vi "UHR-Fleezers Control (host) - 12.7.vi"() -> ()   [LabVIEW 2012] (continued)
                                }
                                frame "4" {
                                n759 = property on="Fl. Triggered..." class="Bool (strict)"("Val(Sgnl)"=TRUE ("Value (Signaling)")) -> ()  [unwired: 2 in, 2 out]
                                }
                                }
                                }
                                }
                                }
                                frame "5", "6" {
                                n760 = stacked-sequence {
                                tunnel: w1212 -> [_ _ _ _ _ _ w1224]
                                frame #0 {
                                n761 = Replace Array Subset(array=u32[] [0] ("Index Values"), new element="Raster Set Upon Tether", index=0) -> (w1213:u32[])
                                n762 = property on="Saved AOD Raster Scan Parameter Sets" class="Arr (strict)"("Index Values"=w1213) -> ()  [unwired: 2 in, 2 out]
                                }
                                frame #1 {
                                n763 = Wait (ms)(milliseconds to wait=u32 500) -> ()  [unwired: 1 out]
                                }
                                frame #2 {
                                n764 = property on="Load parameters" class="Bool (strict)"("Val(Sgnl)"=TRUE ("Value (Signaling)")) -> ()  [unwired: 2 in, 2 out]
                                n765 = case shown="True" "Green ON During Raster" {
                                frame False {
                                }
                                frame True {
                                n766 = property on="Green Laser ON" class="Bool (strict)"("Val(Sgnl)"=TRUE ("Value (Signaling)")) -> ()  [unwired: 2 in, 2 out]
                                }
                                }
                                }
                                frame #3 {
                                n767 = Wait (ms)(milliseconds to wait=u32 500) -> ()  [unwired: 1 out]
                                }
                                frame #4 {
                                n768 = property on="Trap Raster Scan" class="Bool (strict)"("Val(Sgnl)"=TRUE ("Value (Signaling)")) -> ()  [unwired: 2 in, 2 out]
                                }
                                frame #5 {
                                n769 = Wait (ms)(milliseconds to wait=u32 2000) -> ()  [unwired: 1 out]
                                }
                                frame #6 {
                                n770 = flat-sequence {
                                tunnel: w1224 -> [w1231]
                                frame #0 {
                                n771 = while {
                                stop <- w1227 stop-if-true
                                n772 = local read "Raster Scanning..."() -> (w1226:bool)
                                n773 = local read "Saving..."() -> (w1229:bool)
                                n774 = Wait (ms)(milliseconds to wait=u32 100) -> ()  [unwired: 1 out]
                                n775 = Not(x=w1229) -> (.not. x?=w1228:bool)
                                n776 = Not(x=w1226) -> (.not. x?=w1225:bool)
                                n777 = And(x=w1228, y=w1225) -> (x .and. y?=w1227:bool)
                                }
                                }
                                frame #1 {
                                n778 = local read "Tether"() -> (w1232:bool)
                                n779 = case shown="True" w1232 {
                                tunnel: w1231 -> [_ w1234]
                                frame False {
                                n780 = property on="Fish for Tether" class="Bool (strict)"("Val(Sgnl)"="Fish again after \nraster break?") -> ()  [unwired: 2 in, 2 out]
                                }
                                frame True {
                                n781 = stacked-sequence {
                                tunnel: w1234 -> [_ w1238 _ _]
                                frame #0 {
                                n782 = property on="Trap Delta (MHz)" class="DigNum (strict)"("Val(Sgnl)"="Move to Delta 2 (MHz)") -> ()  [unwired: 2 in, 2 out]
                                n783 = case shown="True" "Flow ON after\ntether testing?" {
                                frame False {
                                }
                                frame True {
                                n784 = property on="Sample Channel\nFlow" class="Bool (strict)"("Val(Sgnl)"=TRUE ("Value (Signaling)")) -> ()  [unwired: 2 in, 2 out]
                                }
                                }
                                }
                                frame #1 {
                                n785 = flat-sequence {
                                tunnel: w1238 -> [w1240]
                                frame #0 {
                                n786 = Wait (ms)(milliseconds to wait=u32 500) -> ()  [unwired: 1 out]
                                }
                                frame #1 {
                                n787 = case shown="\"6\"" w1240 {
                                frame Default {
                                }
                                frame "6" {
                                n788 = property on="Green Laser ON" class="Bool (strict)"("Val(Sgnl)"=TRUE ("Green Laser ON/Interlacing")) -> ()  [unwired: 2 in, 2 out]
                                }
                                }
                                }
                                frame #2 {
                                n789 = Wait (ms)(milliseconds to wait=u32 500) -> ()  [unwired: 1 out]
                                }
                                frame #3 {
                                n790 = local write "Start Saving"("Save at end (5, 6)") -> ()
                                }
                                }
                                }
                                frame #2 {
                                n791 = local read "Bead Sep. Int. Time (s)"() -> (w1246:dbl)
                                n792 = Multiply(x=w1246, y=1000.0) -> (x*y=w1245:dbl)
                                n793 = Wait (ms)(milliseconds to wait=w1245) -> ()  [unwired: 1 out]
                                }
                                frame #3 {
                                n794 = property on="Remove Offset" class="Bool (strict)"("Val(Sgnl)"=TRUE ("Value (Signaling)")) -> ()  [unwired: 2 in, 2 out]
                                }
                                }
                                }
                                }
                                }
                                }
                                }
                                }
                                }
                                frame "2", Default {
                                }
                              }
                            }
                          }
                        }
                      }
                      "Tether" <- "Tether Alarm?"
                    }
                  }
                }
                frame #2 {
                  n795 = local read "Oscillate Set 1"() -> (w1253:bool)
                  n796 = local read "Stop All"() -> (w1251:bool)
                  n797 = Or(x=w1253, y=w1248) -> (x .or. y?=w1250:bool)
                  n798 = Not(x=w1250) -> (.not. x?=w1252:bool)
                  n799 = Compound Arithmetic op=OR(w1251, w1252) -> (w1249:bool)
                }
              }
              n800 = node-c288() -> ()  [unwired: 2 out]
            }
            n801 = node-c288(w1085) -> ()  [unwired: 1 out]
          }
        }
      }
      event "Fl. Triggered...": Value Change {
        n802 = event-data() -> ()  [unwired: 7 out]
        n803 = case shown="True" "Fl. Triggered..." {
          frame False {
          }
          frame True {
            n804 = node-c288() -> (w1264:T23)  [unwired: 4 out]
            n805 = timed-loop {
              timing: w1264 -> [_]
              timing-out: [_] -> w1263
              tunnel: "Action" -> [w1272]
              shift-right: [w1269] -> _
              shift-left: u8 255 -> [w1271]
              shift-right: [w1266] -> _
              shift-left: 255 -> [w1268]
              stop <- w1265 stop-if-true
              # "Reset confocal spot"
              n806 = node-c288() -> ()  [unwired: 2 out]
              n807 = flat-sequence {
                tunnel: w1272 -> [w1292]
                tunnel: w1271 -> [w1291]
                tunnel: [w1290] -> w1270
                tunnel: w1268 -> [w1277]
                tunnel: [w1276] -> w1267
                tunnel: [w1671] -> w1265
                tunnel: w1270 -> [w1670]
                tunnel: [w1670] -> w1269
                tunnel: [w1669] -> w1266
                tunnel: w1267 -> [w1669]
                frame #0 {
                  n808 = local read "Delta Fl. 2"() -> (w1289:dbl)
                  n809 = local read "Delta Fl. 1"() -> (w1284:dbl)
                  n810 = Multiply(x="Fl. Delta Thresh. (kHz)", y=1000.0) -> (x*y=w1279:dbl)
                  n811 = Select(t=w1284, s="APD to Watch", f=w1289) -> (s? t:f=w1280:dbl)
                  n812 = Greater?(x=w1280, y=w1279) -> (0:w1285:bool)
                  n813 = Or(x="Force Yank", y=w1285) -> (x .or. y?=w1283:bool)
                  n814 = And(x=w1283, y="Yank when?") -> (x .and. y?=w1281:bool)
                  n815 = case shown="False" w1281 {
                    tunnel: w1292 -> [w1295 w1496]
                    tunnel: w1291 -> [w1297 w1492]
                    tunnel: [w1297 w1490] -> w1290
                    tunnel: w1280 -> [w1303 _]
                    tunnel: w1279 -> [w1302 _]
                    tunnel: "Force Yank" -> [w1300 _]
                    tunnel: w1277 -> [w1299 w1489]
                    tunnel: [w1298 w1489] -> w1276
                    frame False {
                      n816 = Negate(x=w1302) -> (-x=w1294:dbl)
                      n817 = local write "Fl. High"(TRUE ("Fl. High")) -> ()
                      n818 = Less?(x=w1303, y=w1294) -> (x < y?=w1301:bool)
                      n819 = Or(x=w1300, y=w1301) -> (x .or. y?=w1296:bool)
                      n820 = case shown="True" w1296 {
                        tunnel: w1299 -> [w1304 w1314]
                        tunnel: [w1304 w1313] -> w1298
                        tunnel: w1295 -> [_ w1312]
                        frame False {
                        }
                        frame True {
                          n821 = flat-sequence {
                            tunnel: w1314 -> [w1320]
                            tunnel: w1312 -> [w1317]
                            tunnel: [w1319] -> w1311
                            tunnel: [w1318] -> w1310
                            tunnel: [w1317] -> w1309
                            tunnel: w1308 -> [w1316]
                            tunnel: [w1316] -> w1307
                            tunnel: w1306 -> [w1315]
                            tunnel: [w1315] -> w1305
                            tunnel: [w1391] -> w1313
                            tunnel: w1311 -> [w1391]
                            tunnel: w1310 -> [w1390]
                            tunnel: w1309 -> [w1389]
                            tunnel: w1307 -> [w1388]
                            tunnel: w1305 -> [w1387]
                            frame #0 {
                              n822 = call <vilib>:"Beep.vi"() -> ()  [unwired: 12 in]
                              n823 = local write "Waiting"(FALSE ("Waiting")) -> ()
                              n824 = Increment(x=w1320) -> (x+1=w1319:i32)
                              n825 = case shown="\"Image\"" w1317 {
                                tunnel: w1319 -> [_ w1325 _]
                                frame "Alarm", Default {
                                }
                                frame "Yank" {
                                n826 = flat-sequence {
                                tunnel: w1325 -> [w1328]
                                tunnel: [w1327] -> w1324
                                tunnel: [w1326] -> w1323
                                tunnel: w1324 -> [w1338]
                                tunnel: w1323 -> [w1339]
                                frame #0 {
                                n827 = local read "Yank Delay (s)"() -> (w1331:dbl)
                                n828 = local read "N Array El"() -> (w1326:u8)
                                n829 = Quotient & Remainder(x=w1328, y=w1326) -> (x-y*floor(x/y)=w1327:i32)  [unwired: 1 out]
                                n830 = Multiply(x=w1331, y=1000.0) -> (x*y=w1329:dbl)
                                n831 = Wait (ms)(milliseconds to wait=w1329) -> ()  [unwired: 1 out]
                                }
                                frame #1 {
                                n832 = local read "Yank to which?"() -> (w1333:bool)
                                n833 = local read "Random Choice"() -> (w1343:bool)
                                n834 = local read "Yank to Trap Delta (MHz)"() -> (w1336:dbl[])
                                n835 = local read "Yank to SP"() -> (w1337:dbl[])
                                n836 = Random Number (0-1)() -> (number: 0 to 1=w1342:dbl)
                                n837 = Multiply(x=w1339, y=w1342) -> (x*y=w1341:dbl)
                                n838 = Round Toward -Infinity(1:w1341) -> (0:w1340:dbl)
                                n839 = Select(t=w1340, s=w1343, f=w1338) -> (s? t:f=w1334:dbl)
                                n840 = Select(t=w1336, s=w1333, f=w1337) -> (s? t:f=w1335:dbl[])
                                n841 = Index Array(array=w1335, index=w1334) -> (element=w1332:dbl)
                                n842 = case shown="True" w1333 {
                                tunnel: w1332 -> [w1344 w1371]
                                frame False {
                                n843 = flat-sequence {
                                tunnel: w1344 -> [w1345]
                                frame #0 {
                                n844 = property on="Trap Pos FB SP" class="DigNum (strict)"("Val(Sgnl)"=w1345) -> ()  [unwired: 2 in, 2 out]
                                }
                                frame #1 {
                                n845 = Wait (ms)(milliseconds to wait=u32 700) -> ()  [unwired: 1 out]
                                }
                                frame #2 {
                                n846 = local read "Action (%)"() -> (w1350:dbl)
                                n847 = Absolute Value(x=w1350) -> (abs(x)=w1349:dbl)
                                n848 = Greater?(x=w1349, y=70.0) -> (0:w1347:bool)
                                n849 = property on="Remove Action Offset" class="Bool (strict)"("Val(Sgnl)"=w1347) -> ()  [unwired: 2 in, 2 out]
                                }
                                frame #3 {
                                n850 = for {
                                N: 4 -> [_]
                                n851 = flat-sequence {
                                frame #0 {
                                n852 = Wait (ms)(milliseconds to wait=u32 500) -> ()  [unwired: 1 out]
                                }
                                frame #1 {
                                n853 = local read "Action (%)"() -> (w1356:dbl)
                                n854 = Absolute Value(x=w1356) -> (abs(x)=w1355:dbl)
                                n855 = Greater?(x=w1355, y=70.0) -> (0:w1353:bool)
                                n856 = property on="Remove Action Offset" class="Bool (strict)"("Val(Sgnl)"=w1353) -> ()  [unwired: 2 in, 2 out]
                                }
                                }
                                }
                                }
                                frame #4 {
                                n857 = Wait (ms)(milliseconds to wait=u32 500) -> ()  [unwired: 1 out]
                                }
                                frame #5 {
                                n858 = local read "Mean"() -> (w1364:dbl)
                                n859 = Greater?(x=w1364, y=11.0) -> (0:w1358:bool)
                                n860 = Not(x=w1358) -> (.not. x?=w1359:bool)
                                n861 = And(x=w1359, y="Shift confocal") -> (x .and. y?=w1361:bool)
                                n862 = And(x=w1358, y="Shift confocal") -> (x .and. y?=w1362:bool)
                                n863 = case shown="True" w1362 {
                                frame False {
                                }
                                frame True {
                                n864 = local read "Confocal Y 2 (V)"() -> (w1368:dbl)
                                n865 = local read "Confocal X 2 (V)"() -> (w1367:dbl)
                                n866 = property on="AO1" class="Slide (strict)"("Val(Sgnl)"=w1368) -> ()  [unwired: 2 in, 2 out]
                                n867 = property on="AO2" class="Slide (strict)"("Val(Sgnl)"=w1367) -> ()  [unwired: 2 in, 2 out]
                                }
                                }
                                n868 = case shown="True" w1361 {
                                frame False {
                                }
                                frame True {
                                n869 = local read "Confocal Y 1 (V)"() -> (w1366:dbl)
                                n870 = local read "Confocal X 1 (V)"() -> (w1365:dbl)
                                n871 = property on="AO1" class="Slide (strict)"("Val(Sgnl)"=w1366) -> ()  [unwired: 2 in, 2 out]
                                n872 = property on="AO2" class="Slide (strict)"("Val(Sgnl)"=w1365) -> ()  [unwired: 2 in, 2 out]
                                }
                                }
                                }
                                frame #6 {
                                n873 = Wait (ms)(milliseconds to wait=u32 1500) -> ()  [unwired: 1 out]
                                }
                                frame #7 {
                                n874 = property on="Rem fb disp offset" class="Bool (strict)"("Val(Sgnl)"=TRUE ("Value (Signaling)")) -> ()  [unwired: 2 in, 2 out]
                                }
                                }
                                }
                                frame True {
                                n875 = flat-sequence {
                                tunnel: w1371 -> [w1372]
                                frame #0 {
                                n876 = property on="Trap Delta (MHz)" class="DigNum (strict)"("Val(Sgnl)"=w1372) -> ()  [unwired: 2 in, 2 out]
                                }
                                frame #1 {
                                n877 = Wait (ms)(milliseconds to wait=u32 500) -> ()  [unwired: 1 out]
                                }
                                frame #2 {
                                n878 = local read "Shift confocal"() -> (w1378:bool)
                                n879 = local read "Mean"() -> (w1380:dbl)
                                n880 = Greater?(x=w1380, y=11.0) -> (0:w1377:bool)
                                n881 = Not(x=w1377) -> (.not. x?=w1376:bool)
                                n882 = And(x=w1376, y=w1378) -> (x .and. y?=w1374:bool)
                                n883 = And(x=w1377, y=w1378) -> (x .and. y?=w1375:bool)
                                n884 = case shown="True" w1375 {
                                frame False {
                                }
                                frame True {
                                n885 = local read "Confocal Y 2 (V)"() -> (w1384:dbl)
                                n886 = local read "Confocal X 2 (V)"() -> (w1383:dbl)
                                n887 = property on="AO2" class="Slide (strict)"("Val(Sgnl)"=w1383) -> ()  [unwired: 2 in, 2 out]
                                n888 = property on="AO1" class="Slide (strict)"("Val(Sgnl)"=w1384) -> ()  [unwired: 2 in, 2 out]
                                }
                                }
                                n889 = case shown="True" w1374 {
                                frame False {
                                }
                                frame True {
                                n890 = local read "Confocal X 1 (V)"() -> (w1381:dbl)
                                n891 = local read "Confocal Y 1 (V)"() -> (w1382:dbl)
                                n892 = property on="AO2" class="Slide (strict)"("Val(Sgnl)"=w1381) -> ()  [unwired: 2 in, 2 out]
                                n893 = property on="AO1" class="Slide (strict)"("Val(Sgnl)"=w1382) -> ()  [unwired: 2 in, 2 out]
                                }
                                }
                                }
                                }
                                }
                                }
                                }
                                }
                                }
                                frame "Image" {
                                n894 = property on="Confocal Image" class="Bool (strict)"("Val(Sgnl)"=TRUE ("Value (Signaling)")) -> ()  [unwired: 2 in, 2 out]
                                }
                              }
                              n895 = local write "Fl. High"(FALSE ("Fl. High")) -> ()
                              n896 = local read "Time (s)"() -> (w1318:dbl)
                            }
                            frame #1 {
                              n897 = case shown="True" "Auto F Reset" {
                                tunnel: w1390 -> [_ w1395]
                                tunnel: w1389 -> [_ w1394]
                                tunnel: w1388 -> [_ w1393]
                                tunnel: w1387 -> [_ w1392]
                                frame False {
                                }
                                frame True {
                                n898 = node-c288() -> (w1397:T23)  [unwired: 4 in]
                                n899 = timed-loop {
                                timing: w1397 -> [_]
                                timing-out: [_] -> w1396
                                tunnel: w1395 -> [w1402]
                                tunnel: w1394 -> [w1401]
                                tunnel: w1393 -> [w1400]
                                tunnel: w1392 -> [w1399]
                                stop <- w1398 stop-if-true
                                n900 = node-c288() -> ()  [unwired: 1 in, 1 out]
                                n901 = local read "Fl. Delta Thresh. (kHz)"() -> (w1411:dbl)
                                n902 = local read "APD to Watch"() -> (w1412:bool)
                                n903 = local read "Delta Fl. 1"() -> (w1413:dbl)
                                n904 = local read "Delta Fl. 2"() -> (w1414:dbl)
                                n905 = local read "Fl. Triggered..."() -> (w1405:bool)
                                n906 = local read "Stop All"() -> (w1406:bool)
                                n907 = local read "Reset Force"() -> (w1404:bool)
                                n908 = Multiply(x=w1411, y=1000.0) -> (x*y=w1409:dbl)
                                n909 = Select(t=w1413, s=w1412, f=w1414) -> (s? t:f=w1408:dbl)
                                n910 = Not(x=w1405) -> (.not. x?=w1403:bool)
                                n911 = Greater?(x=w1408, y=w1409) -> (0:w1407:bool)
                                n912 = Compound Arithmetic op=OR(w1407, w1406, w1403, w1404) -> (w1398:bool)
                                n913 = case shown="True" w1398 {
                                tunnel: w1402 -> [_ w1418]
                                tunnel: w1401 -> [_ w1422]
                                tunnel: w1400 -> [_ w1421]
                                tunnel: w1399 -> [_ w1420]
                                frame False {
                                }
                                frame True {
                                n914 = case shown="\"Yank\"" w1422 {
                                tunnel: w1421 -> [_ w1432]
                                tunnel: w1420 -> [_ w1430]
                                frame "Image", Default {
                                }
                                frame "Yank" {
                                n915 = flat-sequence {
                                tunnel: [w1435] -> w1433
                                tunnel: w1432 -> [w1435]
                                tunnel: [w1434] -> w1431
                                tunnel: w1430 -> [w1434]
                                tunnel: w1433 -> [w1441]
                                tunnel: w1431 -> [w1439]
                                frame #0 {
                                n916 = local read "Yank Delay (s)"() -> (w1438:dbl)
                                n917 = Multiply(x=w1438, y=1000.0) -> (x*y=w1436:dbl)
                                n918 = Wait (ms)(milliseconds to wait=w1436) -> ()  [unwired: 1 out]
                                }
                                frame #1 {
                                n919 = local read "Yank to which?"() -> (w1440:bool)
                                n920 = case shown="False" w1440 {
                                tunnel: w1441 -> [_ w1469]
                                tunnel: w1439 -> [w1442 _]
                                frame False {
                                n921 = flat-sequence {
                                tunnel: w1442 -> [w1443]
                                frame #0 {
                                n922 = property on="Trap Pos FB SP" class="DigNum (strict)"("Val(Sgnl)"=w1443) -> ()  [unwired: 2 in, 2 out]
                                }
                                frame #1 {
                                n923 = Wait (ms)(milliseconds to wait=u32 700) -> ()  [unwired: 1 out]
                                }
                                frame #2 {
                                n924 = local read "Action (%)"() -> (w1448:dbl)
                                n925 = Absolute Value(x=w1448) -> (abs(x)=w1447:dbl)
                                n926 = Greater?(x=w1447, y=70.0) -> (0:w1445:bool)
                                n927 = property on="Remove Action Offset" class="Bool (strict)"("Val(Sgnl)"=w1445) -> ()  [unwired: 2 in, 2 out]
                                }
                                frame #3 {
                                n928 = for {
                                N: 4 -> [_]
                                n929 = flat-sequence {
                                frame #0 {
                                n930 = Wait (ms)(milliseconds to wait=u32 500) -> ()  [unwired: 1 out]
                                }
                                frame #1 {
                                n931 = local read "Action (%)"() -> (w1454:dbl)
                                n932 = Absolute Value(x=w1454) -> (abs(x)=w1453:dbl)
                                n933 = Greater?(x=w1453, y=70.0) -> (0:w1451:bool)
                                n934 = property on="Remove Action Offset" class="Bool (strict)"("Val(Sgnl)"=w1451) -> ()  [unwired: 2 in, 2 out]
                                }
                                }
                                }
                                }
                                frame #4 {
                                n935 = Wait (ms)(milliseconds to wait=u32 500) -> ()  [unwired: 1 out]
                                }
                                frame #5 {
                                n936 = local read "Shift confocal"() -> (w1459:bool)
                                n937 = local read "Mean"() -> (w1462:dbl)
                                n938 = Greater?(x=w1462, y=11.0) -> (0:w1458:bool)
                                n939 = Not(x=w1458) -> (.not. x?=w1457:bool)
                                n940 = And(x=w1458, y=w1459) -> (x .and. y?=w1460:bool)
                                n941 = And(x=w1457, y=w1459) -> (x .and. y?=w1456:bool)
                                n942 = case shown="True" w1460 {
                                frame False {
                                }
                                frame True {
                                n943 = local read "Confocal X 2 (V)"() -> (w1465:dbl)
                                n944 = local read "Confocal Y 2 (V)"() -> (w1466:dbl)
                                n945 = property on="AO2" class="Slide (strict)"("Val(Sgnl)"=w1465) -> ()  [unwired: 2 in, 2 out]
                                n946 = property on="AO1" class="Slide (strict)"("Val(Sgnl)"=w1466) -> ()  [unwired: 2 in, 2 out]
                                }
                                }
                                n947 = case shown="True" w1456 {
                                frame False {
                                }
                                frame True {
                                n948 = local read "Confocal Y 1 (V)"() -> (w1464:dbl)
                                n949 = local read "Confocal X 1 (V)"() -> (w1463:dbl)
                                n950 = property on="AO1" class="Slide (strict)"("Val(Sgnl)"=w1464) -> ()  [unwired: 2 in, 2 out]
                                n951 = property on="AO2" class="Slide (strict)"("Val(Sgnl)"=w1463) -> ()  [unwired: 2 in, 2 out]
                                }
                                }
                                }
                                frame #6 {
                                n952 = Wait (ms)(milliseconds to wait=u32 1500) -> ()  [unwired: 1 out]
                                }
                                frame #7 {
                                n953 = property on="Rem fb disp offset" class="Bool (strict)"("Val(Sgnl)"=TRUE ("Value (Signaling)")) -> ()  [unwired: 2 in, 2 out]
                                }
                                }
                                }
                                frame True {
                                n954 = flat-sequence {
                                tunnel: w1469 -> [w1470]
                                frame #0 {
                                n955 = property on="Trap Delta (MHz)" class="DigNum (strict)"("Val(Sgnl)"=w1470) -> ()  [unwired: 2 in, 2 out]
                                }
                                frame #1 {
                                n956 = Wait (ms)(milliseconds to wait=u32 500) -> ()  [unwired: 1 out]
                                }
                                frame #2 {
                                n957 = local read "Shift confocal"() -> (w1476:bool)
                                n958 = local read "Mean"() -> (w1477:dbl)
                                n959 = Greater?(x=w1477, y=11.0) -> (0:w1475:bool)
                                n960 = And(x=w1475, y=w1476) -> (x .and. y?=w1473:bool)
                                n961 = Not(x=w1475) -> (.not. x?=w1474:bool)
                                n962 = And(x=w1474, y=w1476) -> (x .and. y?=w1472:bool)
                                n963 = case shown="True" w1473 {
                                frame False {
                                }
                                frame True {
                                n964 = local read "Confocal Y 2 (V)"() -> (w1482:dbl)
                                n965 = local read "Confocal X 2 (V)"() -> (w1481:dbl)
                                n966 = property on="AO1" class="Slide (strict)"("Val(Sgnl)"=w1482) -> ()  [unwired: 2 in, 2 out]
                                n967 = property on="AO2" class="Slide (strict)"("Val(Sgnl)"=w1481) -> ()  [unwired: 2 in, 2 out]
                                }
                                }
                                n968 = case shown="True" w1472 {
                                frame False {
                                }
                                frame True {
                                n969 = local read "Confocal Y 1 (V)"() -> (w1480:dbl)
                                n970 = local read "Confocal X 1 (V)"() -> (w1479:dbl)
                                n971 = property on="AO2" class="Slide (strict)"("Val(Sgnl)"=w1479) -> ()  [unwired: 2 in, 2 out]
                                n972 = property on="AO1" class="Slide (strict)"("Val(Sgnl)"=w1480) -> ()  [unwired: 2 in, 2 out]
                                }
                                }
                                }
                                }
                                }
                                }
                                }
                                }
                                }
                                }
                                n973 = local read "Time (s)"() -> (w1417:dbl)
                                n974 = Subtract(x=w1418, y=w1417) -> (x-y=w1429:dbl)
                                n975 = Number To Decimal String(number=w1429, width (-)=i16 0) -> (decimal integer string=w1427:string)
                                n976 = Concatenate Strings(w1427, " s fluorescence event") -> (w1424:string)
                                n977 = local read "Messages"() -> (w1425:string)
                                n978 = local write "Duration (s)"(w1429) -> ()
                                n979 = call "Update messages.vi"("Message to add"=w1424, "Old message string"=w1425) -> ("New message string"=w1423:string)
                                n980 = local write "Messages"(w1423) -> ()
                                n981 = call <vilib>:"Beep.vi"() -> ()  [unwired: 12 in]
                                n982 = local write "Reset Force"(FALSE ("Force Reset")) -> ()
                                n983 = local write "Fl. High"(TRUE ("Fl. High")) -> ()
                                n984 = local write "Waiting"(TRUE ("Waiting")) -> ()
                                }
                                }
                                n985 = node-c288() -> ()  [unwired: 1 in, 1 out]
                                }
                                n986 = node-c288(w1396) -> ()  [unwired: 1 out]
                                }
                              }
                            }
                          }
                          n987 = local read "Trap Delta (MHz)"() -> (w1308:dbl)
                          n988 = local read "Trap Pos FB SP"() -> (w1306:fxp<+/-,16,1>)
                        }
                      }
                    }
                    frame True {
                      n989 = flat-sequence {
                        tunnel: w1493 -> [w1503]
                        tunnel: [w1503] -> w1497
                        tunnel: w1496 -> [w1502]
                        tunnel: [w1502] -> w1495
                        tunnel: [w1501] -> w1494
                        tunnel: w1492 -> [w1500]
                        tunnel: [w1499] -> w1491
                        tunnel: w1488 -> [w1498]
                        tunnel: [w1498] -> w1487
                        tunnel: w1497 -> [w1573]
                        tunnel: w1495 -> [w1572]
                        tunnel: w1494 -> [w1571]
                        tunnel: w1491 -> [w1570]
                        tunnel: w1487 -> [w1569]
                        tunnel: [w1570] -> w1490
                        frame #0 {
                          n990 = call <vilib>:"Beep.vi"() -> ()  [unwired: 3 in, 9 out]
                          n991 = local write "Waiting"(FALSE ("Waiting")) -> ()
                          n992 = Increment(x=w1500) -> (x+1=w1499:u8)
                          n993 = case shown="\"Yank\"" w1502 {
                            tunnel: w1499 -> [_ _ w1509]
                            frame "Image" {
                              n994 = property on="Confocal Image" class="Bool (strict)"("Val(Sgnl)"=TRUE ("Value (Signaling)")) -> ()  [unwired: 2 in, 2 out]
                            }
                            frame "Alarm", Default {
                            }
                            frame "Yank" {
                              n995 = flat-sequence {
                                tunnel: w1509 -> [w1512]
                                tunnel: [w1511] -> w1508
                                tunnel: ["N Array El"] -> w1507
                                tunnel: w1508 -> [w1526]
                                tunnel: w1507 -> [w1522]
                                frame #0 {
                                n996 = Multiply(x="Yank Delay (s)", y=1000.0) -> (x*y=w1515:dbl)
                                n997 = Quotient & Remainder(x=w1512, y="N Array El") -> (x-y*floor(x/y)=w1511:u8)  [unwired: 1 out]
                                n998 = Wait (ms)(milliseconds to wait=w1515) -> ()  [unwired: 1 out]
                                }
                                frame #1 {
                                n999 = Random Number (0-1)() -> (number: 0 to 1=w1523:dbl)
                                n1000 = Multiply(x=w1522, y=w1523) -> (x*y=w1521:dbl)
                                n1001 = Round Toward -Infinity(1:w1521) -> (0:w1520:dbl)
                                n1002 = Select(t=w1520, s="Random Choice", f=w1526) -> (s? t:f=w1524:dbl)
                                n1003 = Select(t="Yank to Trap Delta (MHz)", s="Yank to which?", f="Yank to SP") -> (s? t:f=w1517:dbl[])
                                n1004 = Index Array(array=w1517, index=w1524) -> (element=w1527:dbl)
                                n1005 = case shown="False" "Yank to which?" {
                                tunnel: w1527 -> [w1528 w1554]
                                frame False {
                                n1006 = flat-sequence {
                                tunnel: w1528 -> [w1529]
                                frame #0 {
                                n1007 = property on="Trap Pos FB SP" class="DigNum (strict)"("Val(Sgnl)"=w1529) -> ()  [unwired: 2 in, 2 out]
                                }
                                frame #1 {
                                n1008 = Wait (ms)(milliseconds to wait=u32 700) -> ()  [unwired: 1 out]
                                }
                                frame #2 {
                                n1009 = local read "Action (%)"() -> (w1534:dbl)
                                n1010 = Absolute Value(x=w1534) -> (abs(x)=w1533:dbl)
                                n1011 = Greater?(x=w1533, y=70.0) -> (0:w1531:bool)
                                n1012 = property on="Remove Action Offset" class="Bool (strict)"("Val(Sgnl)"=w1531) -> ()  [unwired: 2 in, 2 out]
                                }
                                frame #3 {
                                n1013 = for {
                                N: 4 -> [_]
                                n1014 = flat-sequence {
                                frame #0 {
                                n1015 = Wait (ms)(milliseconds to wait=u32 500) -> ()  [unwired: 1 out]
                                }
                                frame #1 {
                                n1016 = local read "Action (%)"() -> (w1540:dbl)
                                n1017 = Absolute Value(x=w1540) -> (abs(x)=w1539:dbl)
                                n1018 = Greater?(x=w1539, y=70.0) -> (0:w1537:bool)
                                n1019 = property on="Remove Action Offset" class="Bool (strict)"("Val(Sgnl)"=w1537) -> ()  [unwired: 2 in, 2 out]
                                }
                                }
                                }
                                }
                                frame #4 {
                                n1020 = local read "Shift confocal"() -> (w1544:bool)
                                n1021 = local read "Mean"() -> (w1547:dbl)
                                n1022 = Greater?(x=w1547, y=11.0) -> (0:w1543:bool)
                                n1023 = Not(x=w1543) -> (.not. x?=w1542:bool)
                                n1024 = And(x=w1542, y=w1544) -> (x .and. y?=w1541:bool)
                                n1025 = And(x=w1543, y=w1544) -> (x .and. y?=w1545:bool)
                                n1026 = case shown="True" w1545 {
                                frame False {
                                }
                                frame True {
                                n1027 = local read "Confocal X 2 (V)"() -> (w1550:dbl)
                                n1028 = local read "Confocal Y 2 (V)"() -> (w1551:dbl)
                                n1029 = property on="AO2" class="Slide (strict)"("Val(Sgnl)"=w1550) -> ()  [unwired: 2 in, 2 out]
                                n1030 = property on="AO1" class="Slide (strict)"("Val(Sgnl)"=w1551) -> ()  [unwired: 2 in, 2 out]
                                }
                                }
                                n1031 = case shown="True" w1541 {
                                frame False {
                                }
                                frame True {
                                n1032 = local read "Confocal X 1 (V)"() -> (w1548:dbl)
                                n1033 = local read "Confocal Y 1 (V)"() -> (w1549:dbl)
                                n1034 = property on="AO1" class="Slide (strict)"("Val(Sgnl)"=w1549) -> ()  [unwired: 2 in, 2 out]
                                n1035 = property on="AO2" class="Slide (strict)"("Val(Sgnl)"=w1548) -> ()  [unwired: 2 in, 2 out]
                                }
                                }
                                }
                                frame #5 {
                                n1036 = Wait (ms)(milliseconds to wait=u32 1500) -> ()  [unwired: 1 out]
                                }
                                frame #6 {
                                n1037 = property on="Rem fb disp offset" class="Bool (strict)"("Val(Sgnl)"=TRUE ("Value (Signaling)")) -> ()  [unwired: 2 in, 2 out]
                                }
                                }
                                }
                                frame True {
                                n1038 = flat-sequence {
                                tunnel: w1554 -> [w1555]
                                frame #0 {
                                n1039 = property on="Trap Delta (MHz)" class="DigNum (strict)"("Val(Sgnl)"=w1555) -> ()  [unwired: 2 in, 2 out]
                                }
                                frame #1 {
                                n1040 = Wait (ms)(milliseconds to wait=u32 500) -> ()  [unwired: 1 out]
                                }
                                frame #2 {
                                n1041 = local read "Shift confocal"() -> (w1559:bool)
                                n1042 = local read "Mean"() -> (w1557:dbl)
                                n1043 = Greater?(x=w1557, y=11.0) -> (0:w1560:bool)
                                n1044 = Not(x=w1560) -> (.not. x?=w1561:bool)
                                n1045 = And(x=w1561, y=w1559) -> (x .and. y?=w1563:bool)
                                n1046 = And(x=w1560, y=w1559) -> (x .and. y?=w1562:bool)
                                n1047 = case shown="True" w1562 {
                                frame False {
                                }
                                frame True {
                                n1048 = local read "Confocal Y 2 (V)"() -> (w1567:dbl)
                                n1049 = local read "Confocal X 2 (V)"() -> (w1566:dbl)
                                n1050 = property on="AO1" class="Slide (strict)"("Val(Sgnl)"=w1567) -> ()  [unwired: 2 in, 2 out]
                                n1051 = property on="AO2" class="Slide (strict)"("Val(Sgnl)"=w1566) -> ()  [unwired: 2 in, 2 out]
                                }
                                }
                                n1052 = case shown="True" w1563 {
                                frame False {
                                }
                                frame True {
                                n1053 = local read "Confocal X 1 (V)"() -> (w1564:dbl)
                                n1054 = local read "Confocal Y 1 (V)"() -> (w1565:dbl)
                                n1055 = property on="AO2" class="Slide (strict)"("Val(Sgnl)"=w1564) -> ()  [unwired: 2 in, 2 out]
                                n1056 = property on="AO1" class="Slide (strict)"("Val(Sgnl)"=w1565) -> ()  [unwired: 2 in, 2 out]
                                }
                                }
                                }
                                }
                                }
                                }
                                }
                              }
                            }
                          }
                          n1057 = local read "Time (s)"() -> (w1501:dbl)
                          "Fl. High" <- TRUE ("Yanking")
                        }
                        frame #1 {
                          n1058 = local read "Auto F Reset"() -> (w1568:bool)
                          n1059 = case shown="True" w1568 {
                            tunnel: w1573 -> [_ w1577]
                            tunnel: w1572 -> [_ w1576]
                            tunnel: w1571 -> [_ w1575]
                            tunnel: w1569 -> [_ w1574]
                            frame False {
                            }
                            frame True {
                              n1060 = node-c288() -> (w1579:T23)  [unwired: 4 out]
                              n1061 = timed-loop {
                                timing: w1579 -> [_]
                                timing-out: [_] -> w1578
                                tunnel: w1577 -> [w1597]
                                tunnel: w1576 -> [w1596]
                                tunnel: w1575 -> [w1595]
                                tunnel: w1574 -> [w1594]
                                stop <- w1580 stop-if-true
                                n1062 = node-c288() -> ()  [unwired: 2 out]
                                n1063 = local read "Fl. Delta Thresh. (kHz)"() -> (w1588:dbl)
                                n1064 = local read "Fl. Triggered..."() -> (w1593:bool)
                                n1065 = local read "Delta Fl. 1"() -> (w1584:dbl)
                                n1066 = local read "Delta Fl. 2"() -> (w1582:dbl)
                                n1067 = local read "Stop All"() -> (w1591:bool)
                                n1068 = local read "APD to Watch"() -> (w1583:bool)
                                n1069 = Select(t=w1584, s=w1583, f=w1582) -> (s? t:f=w1581:dbl)
                                n1070 = Not(x=w1593) -> (.not. x?=w1592:bool)
                                n1071 = Multiply(x=w1588, y=1000.0) -> (x*y=w1587:dbl)
                                n1072 = Negate(x=w1587) -> (-x=w1586:dbl)
                                n1073 = Less?(x=w1581, y=w1586) -> (x < y?=w1590:bool)
                                n1074 = Compound Arithmetic op=OR(w1590, w1591, w1592, "Reset Force") -> (w1580:bool)
                                n1075 = case shown="True" w1580 {
                                tunnel: w1597 -> [_ w1612]
                                tunnel: w1596 -> [_ w1611]
                                tunnel: w1595 -> [_ w1601]
                                tunnel: w1594 -> [_ w1603]
                                frame False {
                                }
                                frame True {
                                n1076 = local read "Time (s)"() -> (w1602:dbl)
                                n1077 = case shown="\"Yank\"" w1611 {
                                tunnel: w1612 -> [_ w1615]
                                tunnel: w1603 -> [_ w1613]
                                frame "Image", Default {
                                }
                                frame "Yank" {
                                n1078 = flat-sequence {
                                tunnel: [w1621] -> w1616
                                tunnel: w1615 -> [w1621]
                                tunnel: [w1617] -> w1614
                                tunnel: w1613 -> [w1617]
                                tunnel: w1616 -> [w1624]
                                tunnel: w1614 -> [w1622]
                                frame #0 {
                                n1079 = local read "Yank Delay (s)"() -> (w1620:dbl)
                                n1080 = Multiply(x=w1620, y=1000.0) -> (x*y=w1618:dbl)
                                n1081 = Wait (ms)(milliseconds to wait=w1618) -> ()  [unwired: 1 out]
                                }
                                frame #1 {
                                n1082 = local read "Yank to which?"() -> (w1623:bool)
                                n1083 = case shown="False" w1623 {
                                tunnel: w1624 -> [_ w1651]
                                tunnel: w1622 -> [w1625 _]
                                frame False {
                                n1084 = flat-sequence {
                                tunnel: w1625 -> [w1626]
                                frame #0 {
                                n1085 = property on="Trap Pos FB SP" class="DigNum (strict)"("Val(Sgnl)"=w1626) -> ()  [unwired: 2 in, 2 out]
                                }
                                frame #1 {
                                n1086 = Wait (ms)(milliseconds to wait=u32 700) -> ()  [unwired: 1 out]
                                }
                                frame #2 {
                                n1087 = local read "Action (%)"() -> (w1631:dbl)
                                n1088 = Absolute Value(x=w1631) -> (abs(x)=w1630:dbl)
                                n1089 = Greater?(x=w1630, y=70.0) -> (0:w1628:bool)
                                n1090 = property on="Remove Action Offset" class="Bool (strict)"("Val(Sgnl)"=w1628) -> ()  [unwired: 2 in, 2 out]
                                }
                                frame #3 {
                                n1091 = for {
                                N: 4 -> [_]
                                n1092 = flat-sequence {
                                frame #0 {
                                n1093 = Wait (ms)(milliseconds to wait=u32 500) -> ()  [unwired: 1 out]
                                }
                                frame #1 {
                                n1094 = local read "Action (%)"() -> (w1637:dbl)
                                n1095 = Absolute Value(x=w1637) -> (abs(x)=w1636:dbl)
                                n1096 = Greater?(x=w1636, y=70.0) -> (0:w1634:bool)
                                n1097 = property on="Remove Action Offset" class="Bool (strict)"("Val(Sgnl)"=w1634) -> ()  [unwired: 2 in, 2 out]
                                }
                                }
                                }
                                }
                                frame #4 {
                                n1098 = local read "Shift confocal"() -> (w1642:bool)
                                n1099 = local read "Mean"() -> (w1644:dbl)
                                n1100 = Greater?(x=w1644, y=11.0) -> (0:w1641:bool)
                                n1101 = Not(x=w1641) -> (.not. x?=w1640:bool)
                                n1102 = And(x=w1641, y=w1642) -> (x .and. y?=w1639:bool)
                                n1103 = And(x=w1640, y=w1642) -> (x .and. y?=w1638:bool)
                                n1104 = case shown="True" w1639 {
                                frame False {
                                }
                                frame True {
                                n1105 = local read "Confocal Y 2 (V)"() -> (w1648:dbl)
                                n1106 = local read "Confocal X 2 (V)"() -> (w1647:dbl)
                                n1107 = property on="AO2" class="Slide (strict)"("Val(Sgnl)"=w1647) -> ()  [unwired: 2 in, 2 out]
                                n1108 = property on="AO1" class="Slide (strict)"("Val(Sgnl)"=w1648) -> ()  [unwired: 2 in, 2 out]
                                }
                                }
                                n1109 = case shown="True" w1638 {
                                frame False {
                                }
                                frame True {
                                n1110 = local read "Confocal X 1 (V)"() -> (w1645:dbl)
                                n1111 = local read "Confocal Y 1 (V)"() -> (w1646:dbl)
                                n1112 = property on="AO1" class="Slide (strict)"("Val(Sgnl)"=w1646) -> ()  [unwired: 2 in, 2 out]
                                n1113 = property on="AO2" class="Slide (strict)"("Val(Sgnl)"=w1645) -> ()  [unwired: 2 in, 2 out]
                                }
                                }
                                }
                                frame #5 {
                                n1114 = Wait (ms)(milliseconds to wait=u32 1500) -> ()  [unwired: 1 out]